vi "FlexMag - 24-03-2023.vi"() -> ()   [LabVIEW 2018] (continued)
                                n22362 = Wait Until Next ms Multiple(millisecond multiple=u32 1000) -> ()  [unwired: 1 out]
                                n22363 = local read "abort ch2"() -> (w26251:bool)
                                n22364 = Decrement(x=w26255) -> (x-1=w26254:dbl)
                                n22365 = local write "time counting"(w26254) -> ()
                                n22366 = Not(x=w26253) -> (.not. x?=w26252:bool)
                                n22367 = Less Or Equal To 0?(x=w26254) -> (x <= 0?=w26250:bool)
                                n22368 = Compound Arithmetic op=OR(w26250, w26252, w26251) -> (w26249:bool)
                                }
                                }
                                }
                                }
                                }
                                }
                                }
                                }
                                frame True {
                                }
                                }
                                }
                                frame #8 {
                                n22369 = local read "abort ch2"() -> (w26256:bool)
                                n22370 = case shown="False" w26256 {
                                frame False {
                                n22371 = local read "coating start"() -> (w26257:bool)
                                n22372 = case shown="True" w26257 {
                                frame False {
                                }
                                frame True {
                                n22373 = local read "R dc step length 9"() -> (w26260:dbl)
                                n22374 = Greater?(x=w26260, y=0.0) -> (0:w26259:bool)
                                n22375 = case shown="True" w26259 {
                                frame False {
                                }
                                frame True {
                                n22376 = flat-sequence {
                                frame #0 {
                                n22377 = local read "R dc step length 9"() -> (w26267:dbl)
                                n22378 = local read "R dc step power 9"() -> (w26262:dbl)
                                n22379 = local read "R web speed"() -> (w26266:dbl)
                                n22380 = Wait (ms)(milliseconds to wait=u32 100) -> ()  [unwired: 1 out]
                                n22381 = Divide(x=w26267, y=w26266) -> (x/y=w26265:dbl)
                                n22382 = local write "Set DC Power ch2"(w26262) -> ()
                                n22383 = Multiply(x=w26265, y=60) -> (x*y=w26263:dbl)
                                n22384 = local write "time counting"(w26263) -> ()
                                }
                                frame #1 {
                                n22385 = local write "Dc_auto_set"(TRUE ("Dc_auto_set")) -> ()
                                }
                                frame #2 {
                                n22386 = while {
                                stop <- w26270 stop-if-true
                                n22387 = local read "time counting"() -> (w26276:dbl)
                                n22388 = local read "coating start"() -> (w26274:bool)
                                n22389 = local read "abort ch2"() -> (w26272:bool)
                                n22390 = Wait Until Next ms Multiple(millisecond multiple=u32 1000) -> ()  [unwired: 1 out]
                                n22391 = Decrement(x=w26276) -> (x-1=w26275:dbl)
                                n22392 = local write "time counting"(w26275) -> ()
                                n22393 = Not(x=w26274) -> (.not. x?=w26273:bool)
                                n22394 = Less Or Equal To 0?(x=w26275) -> (x <= 0?=w26271:bool)
                                n22395 = Compound Arithmetic op=OR(w26271, w26273, w26272) -> (w26270:bool)
                                }
                                }
                                }
                                }
                                }
                                }
                                }
                                }
                                frame True {
                                }
                                }
                                }
                                frame #9 {
                                n22396 = local read "abort ch2"() -> (w26277:bool)
                                n22397 = case shown="False" w26277 {
                                frame False {
                                n22398 = local read "coating start"() -> (w26278:bool)
                                n22399 = case shown="True" w26278 {
                                frame False {
                                }
                                frame True {
                                n22400 = local read "R dc step length 10"() -> (w26281:dbl)
                                n22401 = Greater?(x=w26281, y=0.0) -> (0:w26280:bool)
                                n22402 = case shown="True" w26280 {
                                frame False {
                                }
                                frame True {
                                n22403 = flat-sequence {
                                frame #0 {
                                n22404 = local read "R dc step length 10"() -> (w26288:dbl)
                                n22405 = local read "R dc step power 10"() -> (w26283:dbl)
                                n22406 = local read "R web speed"() -> (w26287:dbl)
                                n22407 = Divide(x=w26288, y=w26287) -> (x/y=w26286:dbl)
                                n22408 = local write "Set DC Power ch2"(w26283) -> ()
                                n22409 = Wait (ms)(milliseconds to wait=u32 100) -> ()  [unwired: 1 out]
                                n22410 = Multiply(x=w26286, y=60) -> (x*y=w26284:dbl)
                                n22411 = local write "time counting"(w26284) -> ()
                                }
                                frame #1 {
                                n22412 = local write "Dc_auto_set"(TRUE ("Dc_auto_set")) -> ()
                                }
                                frame #2 {
                                n22413 = while {
                                stop <- w26291 stop-if-true
                                n22414 = local read "time counting"() -> (w26297:dbl)
                                n22415 = local read "coating start"() -> (w26295:bool)
                                n22416 = local read "abort ch2"() -> (w26293:bool)
                                n22417 = Wait Until Next ms Multiple(millisecond multiple=u32 1000) -> ()  [unwired: 1 out]
                                n22418 = Decrement(x=w26297) -> (x-1=w26296:dbl)
                                n22419 = local write "time counting"(w26296) -> ()
                                n22420 = Not(x=w26295) -> (.not. x?=w26294:bool)
                                n22421 = Less Or Equal To 0?(x=w26296) -> (x <= 0?=w26292:bool)
                                n22422 = Compound Arithmetic op=OR(w26292, w26294, w26293) -> (w26291:bool)
                                }
                                }
                                }
                                }
                                }
                                }
                                }
                                }
                                frame True {
                                }
                                }
                                }
                                frame #10 {
                                n22423 = local read "abort ch2"() -> (w26298:bool)
                                n22424 = case shown="False" w26298 {
                                frame False {
                                n22425 = local read "coating start"() -> (w26299:bool)
                                n22426 = case shown="True" w26299 {
                                frame False {
                                }
                                frame True {
                                n22427 = Wait (ms)(milliseconds to wait=u32 100) -> ()  [unwired: 1 out]
                                "coating ch4 led 12" <- TRUE ("coating ch2 led 1")
                                }
                                }
                                }
                                frame True {
                                }
                                }
                                }
                                }
                                }
                                frame Enabled {
                                n22428 = stacked-sequence {
                                frame #0 {
                                n22429 = local read "abort ch4"() -> (w26302:bool)
                                n22430 = case shown="False" w26302 {
                                frame False {
                                n22431 = local read "coating start"() -> (w26303:bool)
                                n22432 = case shown="True" w26303 {
                                frame False {
                                }
                                frame True {
                                n22433 = flat-sequence {
                                frame #0 {
                                n22434 = local read "R rf step power 1"() -> (w26306:dbl)
                                n22435 = local write "RF_forward_power_1"(w26306) -> ()
                                n22436 = Wait (ms)(milliseconds to wait=u32 100) -> ()  [unwired: 1 out]
                                n22437 = local write "current step"(1.0 ("step up")) -> ()
                                }
                                frame #1 {
                                n22438 = local write "RF_auto_set"(TRUE ("Dc_auto_set")) -> ()
                                }
                                frame #2 {
                                n22439 = Wait (ms)(milliseconds to wait=u32 1000) -> ()  [unwired: 1 out]
                                }
                                }
                                }
                                }
                                }
                                frame True {
                                }
                                }
                                }
                                frame #1 {
                                n22440 = local read "abort ch4"() -> (w26309:bool)
                                n22441 = case shown="False" w26309 {
                                frame False {
                                n22442 = local read "coating start"() -> (w26310:bool)
                                n22443 = case shown="True" w26310 {
                                frame False {
                                }
                                frame True {
                                n22444 = while {
                                i -> [w26311]
                                stop <- w26323 stop-if-true
                                n22445 = local read "step count"() -> (w26326:dbl)
                                n22446 = local read "R RF number steps"() -> (w26324:dbl)
                                n22447 = local read "roll error (min)"() -> (w26314:i32)
                                n22448 = Wait Until Next ms Multiple(millisecond multiple=u32 300) -> ()  [unwired: 1 out]
                                n22449 = feedback #342() -> (w26327:dbl)  [unwired: 1 in]
                                n22450 = feedback-in #342(w26326) -> ()
                                n22451 = Less?(x=w26326, y=w26327) -> (x < y?=w26325:bool)
                                n22452 = Multiply(x=200, y=w26314) -> (x*y=w26313:i32)
                                n22453 = case shown="True" w26325 {
                                tunnel: w26324 -> [_ w26334]
                                tunnel: [FALSE w26331] -> w26317
                                frame False {
                                }
                                frame True {
                                n22454 = local read "current step"() -> (w26333:dbl)
                                n22455 = Greater Or Equal?(x=w26334, y=w26333) -> (x >= y?=w26332:bool)
                                n22456 = Not(x=w26332) -> (.not. x?=w26331:bool)
                                n22457 = case shown="True" w26332 {
                                tunnel: w26333 -> [_ w26335]
                                frame False {
                                }
                                frame True {
                                n22458 = case shown="7" w26335 {
                                frame 0, Default {
                                }
                                frame 1 {
                                n22459 = stacked-sequence {
                                frame #0 {
                                n22460 = local read "R rf step power 1"() -> (w26337:dbl)
                                n22461 = local write "RF_forward_power_1"(w26337) -> ()
                                n22462 = Wait (ms)(milliseconds to wait=u32 100) -> ()  [unwired: 1 out]
                                }
                                frame #1 {
                                n22463 = local write "RF_auto_set"(TRUE ("Dc_auto_set")) -> ()
                                }
                                }
                                }
                                frame 2 {
                                n22464 = stacked-sequence {
                                frame #0 {
                                n22465 = local read "R rf step power 2"() -> (w26340:dbl)
                                n22466 = local write "RF_forward_power_1"(w26340) -> ()
                                n22467 = Wait (ms)(milliseconds to wait=u32 100) -> ()  [unwired: 1 out]
                                }
                                frame #1 {
                                n22468 = local write "RF_auto_set"(TRUE ("Dc_auto_set")) -> ()
                                }
                                }
                                }
                                frame 3 {
                                n22469 = stacked-sequence {
                                frame #0 {
                                n22470 = local read "R rf step power 3"() -> (w26343:dbl)
                                n22471 = local write "RF_forward_power_1"(w26343) -> ()
                                n22472 = Wait (ms)(milliseconds to wait=u32 100) -> ()  [unwired: 1 out]
                                }
                                frame #1 {
                                n22473 = local write "RF_auto_set"(TRUE ("Dc_auto_set")) -> ()
                                }
                                }
                                }
                                frame 4 {
                                n22474 = stacked-sequence {
                                frame #0 {
                                n22475 = local read "R rf step power 4"() -> (w26346:dbl)
                                n22476 = local write "RF_forward_power_1"(w26346) -> ()
                                n22477 = Wait (ms)(milliseconds to wait=u32 100) -> ()  [unwired: 1 out]
                                }
                                frame #1 {
                                n22478 = local write "RF_auto_set"(TRUE ("Dc_auto_set")) -> ()
                                }
                                }
                                }
                                frame 5 {
                                n22479 = stacked-sequence {
                                frame #0 {
                                n22480 = local read "R rf step power 5"() -> (w26349:dbl)
                                n22481 = local write "RF_forward_power_1"(w26349) -> ()
                                n22482 = Wait (ms)(milliseconds to wait=u32 100) -> ()  [unwired: 1 out]
                                }
                                frame #1 {
                                n22483 = local write "RF_auto_set"(TRUE ("Dc_auto_set")) -> ()
                                }
                                }
                                }
                                frame 6 {
                                n22484 = stacked-sequence {
                                frame #0 {
                                n22485 = local read "R rf step power 6"() -> (w26352:dbl)
                                n22486 = local write "RF_forward_power_1"(w26352) -> ()
                                n22487 = Wait (ms)(milliseconds to wait=u32 100) -> ()  [unwired: 1 out]
                                }
                                frame #1 {
                                n22488 = local write "RF_auto_set"(TRUE ("Dc_auto_set")) -> ()
                                }
                                }
                                }
                                frame 7 {
                                n22489 = stacked-sequence {
                                frame #0 {
                                n22490 = local read "R rf step power 7"() -> (w26355:dbl)
                                n22491 = local write "RF_forward_power_1"(w26355) -> ()
                                n22492 = Wait (ms)(milliseconds to wait=u32 100) -> ()  [unwired: 1 out]
                                }
                                frame #1 {
                                n22493 = local write "RF_auto_set"(TRUE ("Dc_auto_set")) -> ()
                                }
                                }
                                }
                                frame 8 {
                                n22494 = stacked-sequence {
                                frame #0 {
                                n22495 = local read "R rf step power 8"() -> (w26358:dbl)
                                n22496 = local write "RF_forward_power_1"(w26358) -> ()
                                n22497 = Wait (ms)(milliseconds to wait=u32 100) -> ()  [unwired: 1 out]
                                }
                                frame #1 {
                                n22498 = local write "RF_auto_set"(TRUE ("Dc_auto_set")) -> ()
                                }
                                }
                                }
                                frame 9 {
                                n22499 = stacked-sequence {
                                frame #0 {
                                n22500 = local read "R rf step power 9"() -> (w26361:dbl)
                                n22501 = local write "RF_forward_power_1"(w26361) -> ()
                                n22502 = Wait (ms)(milliseconds to wait=u32 100) -> ()  [unwired: 1 out]
                                }
                                frame #1 {
                                n22503 = local write "RF_auto_set"(TRUE ("Dc_auto_set")) -> ()
                                }
                                }
                                }
                                frame 10 {
                                n22504 = stacked-sequence {
                                frame #0 {
                                n22505 = local read "R rf step power 10"() -> (w26364:dbl)
                                n22506 = local write "RF_forward_power_1"(w26364) -> ()
                                n22507 = Wait (ms)(milliseconds to wait=u32 100) -> ()  [unwired: 1 out]
                                }
                                frame #1 {
                                n22508 = local write "RF_auto_set"(TRUE ("Dc_auto_set")) -> ()
                                }
                                }
                                }
                                }
                                }
                                }
                                }
                                }
                                n22509 = Greater?(x=w26311, y=w26313) -> (0:w26315:bool)
                                n22510 = case shown="True" w26315 {
                                frame False {
                                }
                                frame True {
                                n22511 = local write "Warning Message"("Automatic Coating Process is canceled !\nCH4  rolling problem..." ("Warning Message")) -> ()
                                n22512 = local write "coating error"(TRUE ("coating error")) -> ()
                                }
                                }
                                n22513 = local read "CH4_Motor DO"() -> (w26319:bool)
                                n22514 = local read "coating start"() -> (w26322:bool)
                                n22515 = local read "abort ch4"() -> (w26320:bool)
                                n22516 = Not(x=w26319) -> (.not. x?=w26318:bool)
                                n22517 = Not(x=w26322) -> (.not. x?=w26321:bool)
                                n22518 = Compound Arithmetic op=OR(w26317, w26318, w26320, w26321) -> (w26323:bool)
                                }
                                }
                                }
                                }
                                frame True {
                                }
                                }
                                }
                                }
                                }
                                }
                                }
                                frame #13 {
                                # "rf off"
                                n22519 = stacked-sequence {
                                frame #0 {
                                n22520 = local read "abort ch4"() -> (w26366:bool)
                                n22521 = case shown="False" w26366 {
                                frame False {
                                n22522 = local read "coating start"() -> (w26367:bool)
                                n22523 = case shown="True" w26367 {
                                frame False {
                                }
                                frame True {
                                n22524 = stacked-sequence {
                                frame #0 {
                                n22525 = Wait (ms)(milliseconds to wait=u32 1000) -> ()  [unwired: 1 out]
                                }
                                frame #1 {
                                n22526 = flat-sequence {
                                frame #0 {
                                n22527 = local write "RF_auto_off"(TRUE ("Dc_auto_off")) -> ()
                                }
                                frame #1 {
                                n22528 = local write "RF_forward_power_1"(i16 0 ("RF_forward_power_1")) -> ()
                                n22529 = Wait (ms)(milliseconds to wait=u32 5000) -> ()  [unwired: 1 out]
                                }
                                frame #2 {
                                n22530 = Wait (ms)(milliseconds to wait=u32 1000) -> ()  [unwired: 1 out]
                                }
                                frame #3 {
                                n22531 = local write "RF_auto_off"(TRUE ("Dc_auto_off")) -> ()
                                }
                                }
                                }
                                }
                                }
                                }
                                }
                                frame True {
                                }
                                }
                                }
                                frame #1 {
                                n22532 = local read "abort ch4"() -> (w26374:bool)
                                n22533 = case shown="False" w26374 {
                                frame False {
                                n22534 = local read "coating start"() -> (w26375:bool)
                                n22535 = case shown="True" w26375 {
                                frame False {
                                }
                                frame True {
                                }
                                }
                                }
                                frame True {
                                }
                                }
                                }
                                frame #2 {
                                n22536 = local read "abort ch4"() -> (w26376:bool)
                                n22537 = case shown="False" w26376 {
                                frame False {
                                n22538 = local read "coating start"() -> (w26377:bool)
                                n22539 = case shown="True" w26377 {
                                frame False {
                                }
                                frame True {
                                n22540 = Wait (ms)(milliseconds to wait=u32 100) -> ()  [unwired: 1 out]
                                "coating ch4 led 13" <- TRUE ("coating ch2 led 1")
                                }
                                }
                                }
                                frame True {
                                }
                                }
                                }
                                }
                                }
                                frame #14 {
                                # "pcgv open"
                                n22541 = stacked-sequence {
                                frame #0 {
                                n22542 = local read "abort ch4"() -> (w26380:bool)
                                n22543 = case shown="False" w26380 {
                                frame False {
                                n22544 = local read "coating start"() -> (w26381:bool)
                                n22545 = case shown="True" w26381 {
                                frame False {
                                }
                                frame True {
                                n22546 = local write "pcgv4 auto open"(TRUE ("ch3 ar set zero auto")) -> ()
                                }
                                }
                                }
                                frame True {
                                }
                                }
                                }
                                frame #1 {
                                n22547 = local read "abort ch4"() -> (w26383:bool)
                                n22548 = case shown="False" w26383 {
                                frame False {
                                n22549 = local read "coating start"() -> (w26384:bool)
                                n22550 = case shown="True" w26384 {
                                frame False {
                                }
                                frame True {
                                n22551 = while {
                                i -> [w26388]
                                stop <- w26390 stop-if-true
                                n22552 = Greater Or Equal?(x=w26388, y=50) -> (x >= y?=w26389:bool)
                                n22553 = case shown="True" w26389 {
                                frame False {
                                }
                                frame True {
                                n22554 = local write "Warning Message"("Automatic Coating Process is canceled !\nCH4 PCGV couldn't be opened..." ("Warning Message")) -> ()
                                n22555 = local write "coating error"(TRUE ("coating error")) -> ()
                                }
                                }
                                n22556 = local read "ch4_pcgv_gui"() -> (w26385:bool)
                                n22557 = case shown="False" w26385 {
                                tunnel: [FALSE ("CH2_WFC_DO") TRUE ("CH2_WFC_DO")] -> w26393
                                frame False {
                                n22558 = Wait Until Next ms Multiple(millisecond multiple=u32 1000) -> ()  [unwired: 1 out]
                                n22559 = local write "pcgv4 auto open"(TRUE ("coating error")) -> ()
                                }
                                frame True {
                                }
                                }
                                n22560 = local read "coating start"() -> (w26392:bool)
                                n22561 = local read "abort ch4"() -> (w26386:bool)
                                n22562 = Not(x=w26392) -> (.not. x?=w26391:bool)
                                n22563 = Compound Arithmetic op=OR(w26393, w26391, w26386) -> (w26390:bool)
                                }
                                }
                                }
                                }
                                frame True {
                                }
                                }
                                }
                                frame #2 {
                                n22564 = local read "abort ch4"() -> (w26400:bool)
                                n22565 = case shown="False" w26400 {
                                frame False {
                                n22566 = local read "coating start"() -> (w26401:bool)
                                n22567 = case shown="True" w26401 {
                                frame False {
                                }
                                frame True {
                                n22568 = Wait (ms)(milliseconds to wait=u32 100) -> ()  [unwired: 1 out]
                                "coating ch4 led 14" <- TRUE ("coating ch2 led 1")
                                }
                                }
                                }
                                frame True {
                                }
                                }
                                }
                                }
                                }
                                frame #15 {
                                # "argon set zero"
                                n22569 = stacked-sequence {
                                frame #0 {
                                n22570 = local read "abort ch4"() -> (w26404:bool)
                                n22571 = case shown="False" w26404 {
                                frame False {
                                n22572 = local read "coating start"() -> (w26405:bool)
                                n22573 = case shown="True" w26405 {
                                frame False {
                                }
                                frame True {
                                n22574 = local write "ch4 ar set zero auto"(TRUE ("ch3 ar set zero auto")) -> ()
                                }
                                }
                                }
                                frame True {
                                }
                                }
                                }
                                frame #1 {
                                n22575 = local read "abort ch4"() -> (w26407:bool)
                                n22576 = case shown="False" w26407 {
                                frame False {
                                n22577 = local read "coating start"() -> (w26408:bool)
                                n22578 = case shown="True" w26408 {
                                frame False {
                                }
                                frame True {
                                n22579 = while {
                                i -> [w26414]
                                stop <- w26416 stop-if-true
                                n22580 = Greater Or Equal?(x=w26414, y=50) -> (x >= y?=w26415:bool)
                                n22581 = case shown="True" w26415 {
                                frame False {
                                }
                                frame True {
                                n22582 = local write "Warning Message"("Automatic Coating Process is canceled !\nCH4 Argon Set Zero problem..." ("Warning Message")) -> ()
                                n22583 = local write "coating error"(TRUE ("coating error")) -> ()
                                }
                                }
                                n22584 = local read "ch4 argon mfc actual"() -> (w26410:dbl)
                                n22585 = Less?(x=w26410, y=1.0) -> (x < y?=w26411:bool)
                                n22586 = case shown="False" w26411 {
                                tunnel: [FALSE ("CH2_WFC_DO") TRUE ("CH2_WFC_DO")] -> w26419
                                frame False {
                                n22587 = Wait Until Next ms Multiple(millisecond multiple=u32 1000) -> ()  [unwired: 1 out]
                                n22588 = local write "ch4 ar set zero auto"(TRUE ("coating error")) -> ()
                                }
                                frame True {
                                }
                                }
                                n22589 = local read "coating start"() -> (w26418:bool)
                                n22590 = local read "abort ch4"() -> (w26412:bool)
                                n22591 = Not(x=w26418) -> (.not. x?=w26417:bool)
                                n22592 = Compound Arithmetic op=OR(w26419, w26417, w26412) -> (w26416:bool)
                                }
                                }
                                }
                                }
                                frame True {
                                }
                                }
                                }
                                frame #2 {
                                n22593 = local read "abort ch4"() -> (w26426:bool)
                                n22594 = case shown="False" w26426 {
                                frame False {
                                n22595 = local read "coating start"() -> (w26427:bool)
                                n22596 = case shown="True" w26427 {
                                frame False {
                                }
                                frame True {
                                n22597 = Wait (ms)(milliseconds to wait=u32 100) -> ()  [unwired: 1 out]
                                "coating ch4 led 15" <- TRUE ("coating ch2 led 1")
                                }
                                }
                                }
                                frame True {
                                }
                                }
                                }
                                }
                                }
                                frame #16 {
                                # "Ar SoV close"
                                n22598 = stacked-sequence {
                                frame #0 {
                                n22599 = local read "abort ch4"() -> (w26430:bool)
                                n22600 = case shown="False" w26430 {
                                frame False {
                                n22601 = local read "coating start"() -> (w26431:bool)
                                n22602 = case shown="True" w26431 {
                                frame False {
                                }
                                frame True {
                                n22603 = while {
                                i -> [w26435]
                                stop <- w26437 stop-if-true
                                n22604 = Greater Or Equal?(x=w26435, y=100) -> (x >= y?=w26436:bool)
                                n22605 = case shown="True" w26436 {
                                frame False {
                                }
                                frame True {
                                n22606 = local write "Warning Message"("Automatic Coating Process is canceled !\nCH4 Argon SoV couldn't be closed..." ("Warning Message")) -> ()
                                n22607 = local write "coating error"(TRUE ("coating error")) -> ()
                                }
                                }
                                n22608 = local read "CH4_SoV_Ar_DI"() -> (w26432:bool)
                                n22609 = case shown="True" w26432 {
                                tunnel: [TRUE ("CH2_WFC_DO") FALSE ("CH2_WFC_DO")] -> w26440
                                frame False {
                                }
                                frame True {
                                n22610 = Wait Until Next ms Multiple(millisecond multiple=u32 200) -> ()  [unwired: 1 out]
                                n22611 = local write "CH4_SoV_Ar_DO"(FALSE ("coating error")) -> ()
                                }
                                }
                                n22612 = local read "coating start"() -> (w26439:bool)
                                n22613 = local read "abort ch4"() -> (w26433:bool)
                                n22614 = Not(x=w26439) -> (.not. x?=w26438:bool)
                                n22615 = Compound Arithmetic op=OR(w26440, w26438, w26433) -> (w26437:bool)
                                }
                                }
                                }
                                }
                                frame True {
                                }
                                }
                                }
                                frame #1 {
                                n22616 = local read "abort ch4"() -> (w26447:bool)
                                n22617 = case shown="False" w26447 {
                                frame False {
                                n22618 = local read "coating start"() -> (w26448:bool)
                                n22619 = case shown="True" w26448 {
                                frame False {
                                }
                                frame True {
                                n22620 = Wait (ms)(milliseconds to wait=u32 100) -> ()  [unwired: 1 out]
                                "coating ch4 led 16" <- TRUE ("coating ch2 led 1")
                                }
                                }
                                }
                                frame True {
                                }
                                }
                                }
                                }
                                }
                                frame #17 {
                                # "BG BV close"
                                n22621 = stacked-sequence {
                                frame #0 {
                                n22622 = local read "abort ch4"() -> (w26451:bool)
                                n22623 = case shown="False" w26451 {
                                frame False {
                                n22624 = local read "coating start"() -> (w26452:bool)
                                n22625 = case shown="True" w26452 {
                                frame False {
                                }
                                frame True {
                                n22626 = while {
                                i -> [w26456]
                                stop <- w26458 stop-if-true
                                n22627 = Greater Or Equal?(x=w26456, y=100) -> (x >= y?=w26457:bool)
                                n22628 = case shown="True" w26457 {
                                frame False {
                                }
                                frame True {
                                n22629 = local write "Warning Message"("Automatic Coating Process is canceled !\nCH4 BG BV couldn't be closed..." ("Warning Message")) -> ()
                                n22630 = local write "coating error"(TRUE ("coating error")) -> ()
                                }
                                }
                                n22631 = local read "CH4_BG_BV_DI"() -> (w26453:bool)
                                n22632 = case shown="True" w26453 {
                                tunnel: [TRUE ("CH2_WFC_DO") FALSE ("CH2_WFC_DO")] -> w26461
                                frame False {
                                }
                                frame True {
                                n22633 = Wait Until Next ms Multiple(millisecond multiple=u32 200) -> ()  [unwired: 1 out]
                                n22634 = local write "CH4_BG_BV_DO"(FALSE ("coating error")) -> ()
                                }
                                }
                                n22635 = local read "coating start"() -> (w26460:bool)
                                n22636 = local read "abort ch4"() -> (w26454:bool)
                                n22637 = Not(x=w26460) -> (.not. x?=w26459:bool)
                                n22638 = Compound Arithmetic op=OR(w26461, w26459, w26454) -> (w26458:bool)
                                }
                                }
                                }
                                }
                                frame True {
                                }
                                }
                                }
                                frame #1 {
                                n22639 = local read "abort ch4"() -> (w26468:bool)
                                n22640 = case shown="False" w26468 {
                                frame False {
                                n22641 = local read "coating start"() -> (w26469:bool)
                                n22642 = case shown="True" w26469 {
                                frame False {
                                }
                                frame True {
                                n22643 = Wait (ms)(milliseconds to wait=u32 100) -> ()  [unwired: 1 out]
                                "coating ch4 led 17" <- TRUE ("coating ch2 led 1")
                                }
                                }
                                }
                                frame True {
                                }
                                }
                                }
                                }
                                }
                                frame #18 {
                                # "CC open"
                                n22644 = stacked-sequence {
                                frame #0 {
                                n22645 = local read "abort ch4"() -> (w26472:bool)
                                n22646 = case shown="False" w26472 {
                                frame False {
                                n22647 = local read "coating start"() -> (w26473:bool)
                                n22648 = case shown="True" w26473 {
                                frame False {
                                }
                                frame True {
                                n22649 = while {
                                i -> [w26477]
                                stop <- w26479 stop-if-true
                                n22650 = Greater Or Equal?(x=w26477, y=100) -> (x >= y?=w26478:bool)
                                n22651 = case shown="True" w26478 {
                                frame False {
                                }
                                frame True {
                                n22652 = local write "Warning Message"("Automatic Coating Process is canceled !\nCH4 CC couldn't be opened..." ("Warning Message")) -> ()
                                n22653 = local write "coating error"(TRUE ("coating error")) -> ()
                                }
                                }
                                n22654 = local read "CH4_CC_DI"() -> (w26474:bool)
                                n22655 = case shown="False" w26474 {
                                tunnel: [FALSE ("CH2_WFC_DO") TRUE ("CH2_WFC_DO")] -> w26482
                                frame False {
                                n22656 = Wait Until Next ms Multiple(millisecond multiple=u32 200) -> ()  [unwired: 1 out]
                                n22657 = local write "CH4_CC_DO"(TRUE ("coating error")) -> ()
                                }
                                frame True {
                                }
                                }
                                n22658 = local read "coating start"() -> (w26481:bool)
                                n22659 = local read "abort ch4"() -> (w26475:bool)
                                n22660 = Not(x=w26481) -> (.not. x?=w26480:bool)
                                n22661 = Compound Arithmetic op=OR(w26482, w26480, w26475) -> (w26479:bool)
                                }
                                }
                                }
                                }
                                frame True {
                                }
                                }
                                }
                                frame #1 {
                                n22662 = local read "abort ch4"() -> (w26489:bool)
                                n22663 = case shown="False" w26489 {
                                frame False {
                                n22664 = local read "coating start"() -> (w26490:bool)
                                n22665 = case shown="True" w26490 {
                                frame False {
                                }
                                frame True {
                                n22666 = Wait (ms)(milliseconds to wait=u32 100) -> ()  [unwired: 1 out]
                                "coating ch4 led 18" <- TRUE ("coating ch2 led 1")
                                }
                                }
                                }
                                frame True {
                                }
                                }
                                }
                                }
                                }
                                frame #19 {
                                # "water close"
                                n22667 = stacked-sequence {
                                frame #0 {
                                n22668 = local read "abort ch4"() -> (w26493:bool)
                                n22669 = case shown="False" w26493 {
                                frame False {
                                n22670 = local read "coating start"() -> (w26494:bool)
                                n22671 = case shown="True" w26494 {
                                frame False {
                                }
                                frame True {
                                n22672 = while {
                                i -> [w26498]
                                stop <- w26500 stop-if-true
                                n22673 = Greater Or Equal?(x=w26498, y=100) -> (x >= y?=w26499:bool)
                                n22674 = case shown="True" w26499 {
                                frame False {
                                }
                                frame True {
                                n22675 = local write "Warning Message"("Automatic Coating Process is canceled !\nCH4 Water Flow couldn't be closed..." ("Warning Message")) -> ()
                                n22676 = local write "coating error"(TRUE ("coating error")) -> ()
                                }
                                }
                                n22677 = local read "CH4_WFC_DI"() -> (w26495:bool)
                                n22678 = case shown="True" w26495 {
                                tunnel: [TRUE ("CH2_WFC_DO") FALSE ("CH2_WFC_DO")] -> w26503
                                frame False {
                                }
                                frame True {
                                n22679 = Wait Until Next ms Multiple(millisecond multiple=u32 200) -> ()  [unwired: 1 out]
                                n22680 = local write "CH4_WFC_DO"(FALSE ("coating error")) -> ()
                                }
                                }
                                n22681 = local read "coating start"() -> (w26502:bool)
                                n22682 = local read "abort ch4"() -> (w26496:bool)
                                n22683 = Not(x=w26502) -> (.not. x?=w26501:bool)
                                n22684 = Compound Arithmetic op=OR(w26503, w26501, w26496) -> (w26500:bool)
                                }
                                }
                                }
                                }
                                frame True {
                                }
                                }
                                }
                                frame #1 {
                                n22685 = local read "abort ch4"() -> (w26510:bool)
                                n22686 = case shown="False" w26510 {
                                frame False {
                                n22687 = local read "coating start"() -> (w26511:bool)
                                n22688 = case shown="True" w26511 {
                                frame False {
                                }
                                frame True {
                                n22689 = Wait (ms)(milliseconds to wait=u32 100) -> ()  [unwired: 1 out]
                                "coating ch4 led 19" <- TRUE ("coating ch2 led 1")
                                }
                                }
                                }
                                frame True {
                                }
                                }
                                }
                                }
                                }
                                frame #20 {
                                # "back roll"
                                n22690 = stacked-sequence {
                                frame #0 {
                                n22691 = local read "abort ch4"() -> (w26514:bool)
                                n22692 = case shown="False" w26514 {
                                frame False {
                                n22693 = local read "coating start"() -> (w26515:bool)
                                n22694 = case shown="True" w26515 {
                                frame False {
                                }
                                frame True {
                                n22695 = disable-structure shown="Enabled" {
                                frame Disabled {
                                n22696 = flat-sequence {
                                frame #0 {
                                n22697 = local read "R RF number steps"() -> (w26516:dbl)
                                n22698 = local write "step count"(w26516) -> ()
                                n22699 = local write "back roll"(TRUE ("back roll")) -> ()
                                }
                                frame #1 {
                                n22700 = Wait (ms)(milliseconds to wait=u32 1000) -> ()  [unwired: 1 out]
                                }
                                frame #2 {
                                n22701 = while {
                                stop <- w26524 stop-if-true
                                n22702 = local read "coating start"() -> (w26521:bool)
                                n22703 = local read "back roll"() -> (w26520:bool)
                                n22704 = local read "abort ch4"() -> (w26523:bool)
                                n22705 = Not(x=w26520) -> (.not. x?=w26519:bool)
                                n22706 = Not(x=w26521) -> (.not. x?=w26525:bool)
                                n22707 = Compound Arithmetic op=OR(w26519, w26525, w26523) -> (w26524:bool)
                                n22708 = Wait Until Next ms Multiple(millisecond multiple=u32 200) -> ()  [unwired: 1 out]
                                }
                                }
                                }
                                }
                                frame Enabled {
                                n22709 = local read "dep. for?"() -> (w26527:bool)
                                n22710 = Not(x=w26527) -> (.not. x?=w26528:bool)
                                n22711 = Wait (ms)(milliseconds to wait=u32 100) -> ()  [unwired: 1 out]
                                n22712 = local write "dep. for?"(w26528) -> ()
                                }
                                }
                                }
                                }
                                }
                                frame True {
                                }
                                }
                                }
                                frame #1 {
                                n22713 = local read "abort ch4"() -> (w26529:bool)
                                n22714 = case shown="False" w26529 {
                                frame False {
                                n22715 = local read "coating start"() -> (w26530:bool)
                                n22716 = case shown="True" w26530 {
                                frame False {
                                }
                                frame True {
                                n22717 = Wait (ms)(milliseconds to wait=u32 100) -> ()  [unwired: 1 out]
                                "coating ch4 led 20" <- TRUE ("coating ch2 led 1")
                                }
                                }
                                }
                                frame True {
                                }
                                }
                                }
                                }
                                }
                                frame #21 {
                                # "done"
                                n22718 = stacked-sequence {
                                frame #0 {
                                n22719 = local read "abort ch4"() -> (w26533:bool)
                                n22720 = case shown="False" w26533 {
                                frame False {
                                n22721 = local read "coating start"() -> (w26534:bool)
                                n22722 = case shown="True" w26534 {
                                frame False {
                                }
                                frame True {
                                n22723 = local write "Buzzer DO"(TRUE ("Buzzer DO")) -> ()
                                n22724 = Wait (ms)(milliseconds to wait=u32 3000) -> ()  [unwired: 1 out]
                                n22725 = local write "System Status"("COATING PROCESS DONE (CH4)" ("System Status")) -> ()
                                }
                                }
                                }
                                frame True {
                                }
                                }
                                }
                                frame #1 {
                                n22726 = local read "abort ch4"() -> (w26538:bool)
                                n22727 = case shown="False" w26538 {
                                frame False {
                                n22728 = local read "coating start"() -> (w26539:bool)
                                n22729 = case shown="True" w26539 {
                                frame False {
                                }
                                frame True {
                                n22730 = Wait (ms)(milliseconds to wait=u32 1000) -> ()  [unwired: 1 out]
                                n22731 = local write "System Status"("SEMI-AUTOMATIC MODE " ("System Status")) -> ()
                                n22732 = local write "Buzzer DO"(FALSE ("Buzzer DO")) -> ()
                                }
                                }
                                }
                                frame True {
                                }
                                }
                                }
                                }
                                }
                                }
                                }
                              }
                            }
                          }
                        }
                        frame 1 {
                          # "MULTILAYER PROCESS"
                        }
                      }
                    }
                  }
                }
                frame True {
                  # "process done OR wrong file"
                  n22733 = local read "coating process done"() -> (w26543:bool)